vi "UHR-Fleezers Control (host) - Avogadro v1.vi"() -> ()   [LabVIEW 2014] (continued)
              }
            }
          }
          frame "Do nothing" {
          }
          frame "Initialize", Default {
            n3430 = Increment(x=w4831) -> (x+1=w4835:i32)
            n3431 = Select(t=1, s=w4824, f=w4835) -> (s? t:f=w4825:i32)
            n3432 = feedback #20(w4833) -> (w4839:dbl[])
            n3433 = Build Array (concatenate)(w4833, w4839) -> (w4832:dbl[])
            n3434 = Greater Or Equal?(x=w4825, y="Wait to get offset (n)") -> (x >= y?=w4828:bool)
            n3435 = Select(t=w4833, s=w4824, f=w4832) -> (s? t:f=w4834:dbl[])
            n3436 = feedback-in #20(w4834) -> ()
            n3437 = call-poly <vilib>:"Mean.vi"("X"=w4834) -> ("mean"=w4829:dbl)  [unwired: 1 out]
            n3438 = local write "Mean T1 Position\nto compare (nm)"(w4829) -> ()
            n3439 = case shown="True" w4824 {
              tunnel: w4827 -> [_ w4845]
              tunnel: w4826 -> [_ w4844]
              frame False {
              }
              frame True {
                w4841 = FALSE ("FPGA Trap Trig")
                n3440 = xnode "Read/Write Control"("FPGA VI Reference In"=w4845, "error in"=w4844, "FPGA Trap Trig"=w4841) -> ("FPGA VI Reference Out"=w4843:T41, "error out"=w4842:errorcluster)
                n3441 = xnode "Read/Write Control"("FPGA VI Reference In"=w4843, "error in"=w4842, "TTrig?"=w4841) -> ()  [unwired: 2 out]
              }
            }
            n3442 = Select(t="Wait for trigger", s=w4828, f="Initialize") -> (s? t:f=w4836:string)
            n3443 = case shown="True" w4828 {
              tunnel: w4829 -> [_ w4848]
              tunnel: w4827 -> [_ w4857]
              tunnel: w4826 -> [_ w4856]
              frame False {
                n3444 = local write "Waiting"(FALSE ("Waiting")) -> ()
                "Initializing" <- TRUE ("Initializing")
              }
              frame True {
                n3445 = local read "Threshold (nm)"() -> (w4860:dbl)
                n3446 = local read "AOM X Cal (nm/MHz)"() -> (w4859:dbl)
                n3447 = Add(x=w4848, y=w4860) -> (x+y=w4861:dbl)
                n3448 = Divide(x=w4861, y=w4859) -> (x/y=w4858:dbl)
                n3449 = call "IR AOM freq to word.vi"("Frequency In (MHz)"=w4858) -> ("Frequency Word Out (double)"=w4855:dbl)
                n3450 = local write "Initializing"(FALSE ("Initializing")) -> ()
                n3451 = local write "Waiting"(TRUE ("Waiting")) -> ()
                n3452 = To Quad Integer(1:w4855) -> (0:w4854:i64)
                n3453 = xnode "Read/Write Control"("FPGA VI Reference In"=w4857, "error in"=w4856, "FPGA TTrig Thresh"=w4854) -> ("FPGA VI Reference Out"=w4851:T41, "error out"=w4850:errorcluster)
                n3454 = xnode "Read/Write Control"("FPGA VI Reference In"=w4851, "error in"=w4850, "FPGA Trap Trig"=TRUE) -> ()  [unwired: 2 out]
              }
            }
          }
        }
      }
    }
    n3455 = feedback-in #18(w4440) -> ()
    n3456 = feedback-in #19(w4437) -> ()
    n3457 = xnode ("Read/Write Control")("FPGA VI Reference In"=w4251, "error in"=w4523) -> ("FPGA VI Reference Out"=w4325:T41, "error out"=w4425:errorcluster, "AI2 Y Sum Set 1"=w4572:i16, "AI2 Y Sum Set 2"=w4571:i16, "AI1 X Set 1"=w4463:fxp<+/-,16,1>, "AI1 X Set 2"=w4462:fxp<+/-,16,1>, "Trap Pos FB Int Signal"=→"Trap Pos FB Int Signal":fxp<+/-,24,9>, "Trap Pos FB Int-Norm Signal"=→"Trap Pos FB Int-Norm Signal":fxp<+/-,16,1>, "Trap Pos FB Action"=w4456:i64, "Scanning"=→"AOD Scanning":bool, "Scan I"=→"AOD Scan I":u64, "Scanning MCL"=w4574:bool, "Scan I (MCL)"=→"MCL Scan I":u64, "Green FB Sum"=w4536:i16, "Trap Pos FB Action"=w4423:i64, "TTrig Fin Thresh"=w4419:i64, "Red FB Intensity"=w4406:i16, "Blue Intensity"=w4401:i16, "BD1 Frequency Out 1"=w4342:u64)
    "MCL Scanning" <- w4574
    "Trap Pos FB Action" <- w4456
    n3458 = Divide(x=w4406, y=3276.7) -> (x/y=w4405:dbl)
    "Red laser intensity (V)" <- w4405
    n3459 = Divide(x=w4401, y=3276.7) -> (x/y=w4400:dbl)
    "Blue laser intensity (V)" <- w4400
    n3460 = Divide(x=w4536, y=3276.7) -> (x/y=w4404:dbl)
    "Green laser intensity (V)" <- w4404
    n3461 = local read "FB Trig Integrate"() -> (w4417:u32)
    n3462 = Divide(x=w4423, y=w4417) -> (x/y=w4416:dbl)
    "TTrig Sig (Int)" <- w4416
    n3463 = Bundle(w4404, w4405, w4400) -> (→"Fluorescence laser intensities plot":cluster{dbl, dbl, dbl})  [unwired: 1 in]
    n3464 = Divide(x=w4419, y=w4417) -> (x/y=w4414:dbl)
    "TTrig Fin Thresh (Int)" <- w4414
    n3465 = local read "AOM X Cal (nm/MHz)"() -> (w4422:dbl)
    n3466 = local read "AI2 (V)"() -> (w4573:cluster{"Set 1":dbl, "Set 2":dbl})
    n3467 = Bundle By Name(cluster=w4573, "Set 1"=w4572, "Set 2"=w4571) -> (w4344:cluster{"Set 1":dbl, "Set 2":dbl})
    n3468 = Divide(x=w4456, y=327.67) -> (x/y=→"Action (%)":dbl)
    n3469 = case shown="True" "Semi Passive Mode" {
      tunnel: w4323 -> [_ w4638]
      frame False {
      }
      frame True {
        n3470 = local read "Target Force (pN)"() -> (w4636:dbl)
        n3471 = Less?(x="Jump Force (pN)", y=w4636) -> (x < y?=w4634:bool)
        n3472 = case shown="False" w4634 {
          tunnel: "Jump Force (pN)" -> [w4644 w4647]
          tunnel: w4638 -> [w4643 w4646]
          tunnel: [w4642 w4645] -> w4637
          frame False {
            n3473 = Less?(x=w4644, y=w4643) -> (x < y?=w4642:bool)
          }
          frame True {
            n3474 = Greater?(x=w4647, y=w4646) -> (0:w4645:bool)
          }
        }
        n3475 = case shown="False" w4637 {
          frame False {
            n3476 = local read "Trap Pos. FB ON"() -> (w4639:bool)
            n3477 = case shown="False" w4639 {
              frame False {
              }
              frame True {
                n3478 = property on="Trap Pos. FB ON" class="Bool (strict)"("Val(Sgnl)"=FALSE) -> ()  [unwired: 2 in, 2 out]
              }
            }
          }
          frame True {
            n3479 = property on="Trap Pos. FB ON" class="Bool (strict)"("Val(Sgnl)"=TRUE) -> ()  [unwired: 2 in, 2 out]
          }
        }
      }
    }
    n3480 = local read "Trap X (AI1)"() -> (w4476:T15)
    n3481 = call "IR AOM word double to freq.vi"("Frequency Word In (double)"=w4414) -> ("Frequency Out (MHz)"=w4413:dbl)
    n3482 = call "IR AOM word double to freq.vi"("Frequency Word In (double)"=w4416) -> ("Frequency Out (MHz)"=w4415:dbl)
    n3483 = Divide(x=w4344, y=3276.7) -> (x/y=w4569:cluster{"Set 1":dbl, "Set 2":dbl})
    n3484 = Multiply(x=w4415, y=w4422) -> (x*y=w4421:dbl)
    "TTrig Sig (nm)" <- w4421
    n3485 = Multiply(x=w4413, y=w4422) -> (x*y=w4420:dbl)
    "TTrig Fin Thresh (nm)" <- w4420
    n3486 = local write "AI2 (V)"(w4569) -> ()
    n3487 = Bundle(cluster=w4476, "Trap 1"=w4463, "Trap 2"=w4462) -> (→"Trap X (AI1)":T15)
    n3488 = local read "Trap Pos. FB ON"() -> (w4330:bool)
    n3489 = local read "Dynamic Force FB (ronen)"() -> (w4331:bool)
    n3490 = Bundle(w4421, w4420) -> (→"TTrig":cluster{dbl, dbl})  [unwired: 1 in]
    n3491 = Compound Arithmetic op=AND(w4331, "Real time Offset file correction for setpoint", w4330) -> (w4332:bool)
    n3492 = case shown="True" w4332 {
      tunnel: w4342 -> [_ _]
      tunnel: w4328 -> [_ w4666]
      tunnel: w4325 -> [_ w4649]
      frame False {
      }
      frame True {
        # "Changed by Ronen - real time update of set point\naccording to offset file"
        n3493 = local read "T1 calibration"() -> (w4661:T9)
        n3494 = local read "Offset file step size"() -> (w4668:dbl)
        n3495 = local read "Setpoint offset\ncorrection values"() -> (w4665:dbl[])
        n3496 = Multiply(x="Target Force (pN)", y=2.0) -> (x*y=w4662:dbl)
        n3497 = local read "Negate Diff?"() -> (w4650:bool)
        n3498 = Unbundle By Name(w4661) -> ("alpha_x (nm/V)"=w4660:dbl, "kappa_x (pN/nm)"=w4659:dbl)
        n3499 = Divide(x=w4666, y=w4668) -> (x/y=w4669:dbl)
        n3500 = To Long Integer(number=w4669) -> (32bit integer=w4667:i32)
        n3501 = Index Array(array=w4665, index=w4667) -> (element=w4652:dbl)
        n3502 = Multiply(x=w4660, y=w4659) -> (x*y=w4658:dbl)
        n3503 = Select(t=1, s=w4650, f=-1) -> (s? t:f=w4653:i32)
        n3504 = Divide(x=w4662, y=w4658) -> (x/y=w4657:dbl)
        n3505 = Multiply(x=w4653, y=w4652) -> (x*y=w4651:dbl)
        n3506 = Add(x=w4657, y=w4651) -> (x+y=w4656:dbl)
        n3507 = To Fixed-Point(number=w4656) -> (fixed-point=w4648:fxp<+/-,16,1>)  [unwired: 1 in]
        "Actual Setpoint" <- w4648
        n3508 = xnode "Read/Write Control"("FPGA VI Reference In"=w4649, "Trap Pos. FB SP"=w4648) -> ()  [unwired: 1 in, 2 out]
      }
    }
    n3509 = local read "All FB On/Off"() -> (w4343:bool)
    n3510 = case shown="True" w4343 {
      tunnel: w4344 -> [_ w4672]
      frame False {
      }
      frame True {
        n3511 = Divide(x=w4672, y=3276.7) -> (x/y=w4670:cluster{"Set 1":dbl, "Set 2":dbl})
        n3512 = Unbundle By Name(w4670) -> ("Set 1"=w4677:dbl, "Set 2"=w4676:dbl)
        n3513 = Greater?(x=w4677, y="Feedback Auto-Off threshold") -> (0:w4675:bool)
        n3514 = Greater?(x=w4676, y="Feedback Auto-Off threshold") -> (0:w4674:bool)
        n3515 = Or(x=w4675, y=w4674) -> (x .or. y?=w4673:bool)
        n3516 = case shown="True" w4673 {
          frame False {
          }
          frame True {
            n3517 = property on="All FB On/Off" class="Bool (strict)"("Val(Sgnl)"=FALSE) -> ()  [unwired: 2 in, 2 out]
          }
        }
      }
    }
    n3518 = flat-sequence "To save data" {
      tunnel: [w5430] -> w4592
      tunnel: [w5431] -> w4591
      tunnel: w4554 -> [w5424]
      tunnel: w4284 -> [w5428]
      tunnel: ["Save Calibration"] -> w4566
      tunnel: w4314 -> [w5427]
      tunnel: [w5420] -> w4563
      tunnel: [w5417] -> w4562
      tunnel: [w5414] -> w4561
      tunnel: w4553 -> [w5416]
      tunnel: w4250 -> [w5410]
      tunnel: [w5410] -> w4517
      tunnel: ["Start Saving"] -> w4497
      tunnel: [w5405] -> w4446
      tunnel: [w5404] -> w4445
      tunnel: [w5401] -> w4348
      tunnel: [w5397] -> w4336
      tunnel: w4592 -> [w5742]
      tunnel: w4591 -> [w5741]
      tunnel: w4315 -> [w5740]
      tunnel: w4566 -> [w5739]
      tunnel: w4563 -> [w5737]
      tunnel: w4562 -> [w5736]
      tunnel: w4561 -> [w5735]
      tunnel: w4307 -> [w5734]
      tunnel: w4313 -> [w5733]
      tunnel: w4517 -> [w5732]
      tunnel: w4497 -> [w5731]
      tunnel: w4355 -> [w5730]
      tunnel: w4396 -> [w5729]
      tunnel: w4446 -> [w5728]
      tunnel: w4445 -> [w5727]
      tunnel: w4444 -> [w5726]
      tunnel: w4256 -> [w5725]
      tunnel: w4312 -> [w5724]
      tunnel: w4348 -> [w5723]
      tunnel: w4336 -> [w5722]
      frame #0 {
        # "Changed by Ronen - we don't have a database so we disabled this"
        n3519 = Or(x="Save N Sets", y="Start Saving") -> (x .or. y?=w5411:bool)
        n3520 = To Double Precision Float(number=w5427) -> (double precision float=w5421:dbl)
        n3521 = Build Array(w5411, "Save Calibration", w5424, w5416, "Flow Cal") -> (w5426:bool[])
        n3522 = Compound Arithmetic op=OR("Save Calibration", w5424, w5411, w5416, "Flow Cal") -> (w5429:bool)
        n3523 = Boolean Array To Number(Boolean array=w5426) -> (number=w5423:u32)
        n3524 = feedback #21(FALSE ("Save APD Data\nwith Trap Data")) -> (w5406:bool)
        n3525 = feedback #22(refnum<k0> refnum) -> (w5432:refnum<file>)
        n3526 = feedback #23(FALSE ("Save APD Data\nwith Trap Data")) -> (w5415:bool)
        n3527 = feedback #24(0) -> (w5434:i32)
        n3528 = feedback #25() -> (w5422:u32)  [unwired: 1 out]
        n3529 = feedback #26(refnum<k0> refnum) -> (w5402:refnum<file>)
        n3530 = feedback #27(refnum<k0> refnum) -> (w5408:refnum<file>)
        n3531 = feedback #28(refnum<k0> refnum) -> (w5398:refnum<file>)
        n3532 = feedback #29(refnum<k0> refnum) -> (w5418:refnum<file>)
        n3533 = case shown="True" w5429 {
          tunnel: [w5443 1] -> w5430
          tunnel: w5434 -> [w5445 _]
          tunnel: [w5444 w5477] -> w5431
          tunnel: w5432 -> [w5444 _]
          tunnel: w5428 -> [_ w5495]
          tunnel: w5421 -> [_ w5493]
          tunnel: w5423 -> [_ w5496]
          tunnel: [w5442 w5476] -> w5420
          tunnel: w5422 -> [w5442 _]
          tunnel: [w5441 w5474] -> w5417
          tunnel: w5418 -> [w5441 _]
          tunnel: [w5440 w5473] -> w5414
          tunnel: w5415 -> [w5440 _]
          tunnel: "Start Saving" -> [_ w5471]
          tunnel: w5410 -> [_ w5470]
          tunnel: [w5439 w5463] -> w5404
          tunnel: w5408 -> [w5439 _]
          tunnel: [w5438 w5462] -> w5405
          tunnel: w5406 -> [w5438 _]
          tunnel: [w5437 w5448] -> w5401
          tunnel: w5402 -> [w5437 _]
          tunnel: [w5436 w5446] -> w5397
          tunnel: w5398 -> [w5436 _]
          frame False {
            n3534 = Increment(x=w5445) -> (x+1=w5443:i32)
          }
          frame True {
            w5447 = FALSE ("Start Saving")
            w5472 = 10.0  # File Version
            w5479 = FALSE ("prepend array or string size? (T)")
            w5478 = T45."big-endian, network order" ("byte order (0:big-endian, network order)")
            # "Ronen Changed the create file - changed data folder to c:\\Data"
            # "Save trap position\ndata"
            n3535 = Array Size(array=w5470) -> (size(s)=w5469:i32)
            n3536 = To Double Precision Float(number=w5469) -> (double precision float=w5468:dbl)
            n3537 = local read "BD 1 Frequency 1 (MHz)"() -> (w5492:dbl)
            n3538 = local read "BD 2 Frequency 1 (MHz)"() -> (w5491:dbl)
            n3539 = local read "BD 1 Frequency 2 (MHz)"() -> (w5490:dbl)
            n3540 = local read "BD 2 Frequency 2 (MHz)"() -> (w5489:dbl)
            n3541 = local read "BD 1 Frequency 3 (MHz)"() -> (w5488:dbl)
            n3542 = local read "BD 2 Frequency 3 (MHz)"() -> (w5487:dbl)
            n3543 = local write "Flow Cal"(w5447) -> ()
            n3544 = local write "Save Calibration"(w5447) -> ()
            n3545 = local write "Start Saving"(w5447) -> ()
            n3546 = Build Array("Save APD Data\nwith Trap Data", "Save Trap Pos. Data") -> (w5465:bool[])
            n3547 = Boolean Array To Number(Boolean array=w5465) -> (number=w5464:u32)
            n3548 = Build Array(w5492, w5491, w5490, w5489, w5488, w5487) -> (w5486:dbl[])
            n3549 = case shown="4" w5496 {
              tunnel: w5495 -> [w5596 w5623 w5639 w5677 w5714]
              tunnel: w5468 -> [w5601 w5630 w5659 w5696 w5719]
              tunnel: w5493 -> [w5600 w5629 w5658 w5695 w5718]
              tunnel: [w5597 w5625 w5650 w5687 w5715] -> w5484
              tunnel: [w5588 "Cal sets to save" w5640 w5678 w5701] -> w5476
              tunnel: w5486 -> [w5598 w5626 w5652 w5689 w5716]
              tunnel: "Save APD Data\nwith Trap Data" -> [w5595 w5612 w5636 w5675 w5713]
              tunnel: [w5595 w5610 w5636 w5675 w5713] -> w5473
              tunnel: w5472 -> [w5591 w5619 w5634 w5673 w5709]
              tunnel: w5471 -> [w5590 _ _ _ _]
              tunnel: [w5581 w5618 w5633 w5663 w5708] -> w5462
              tunnel: "Save Trap Pos. Data" -> [w5581 w5617 w5633 w5663 w5708]
              tunnel: w5464 -> [w5580 w5616 w5632 w5662 w5707]
              frame 1, Default {
                # "timeseries"
                n3550 = case shown="True" "Profile" {
                  tunnel: [w5604 w5608] -> w5585
                  tunnel: [w5604 w5607] -> w5584
                  tunnel: [w5604 w5606] -> w5583
                  tunnel: [w5604 w5605] -> w5582
                  frame False {
                    w5604 = 0.0 ("f")
                  }
                  frame True {
                    n3551 = local read "Current Position"() -> (w5609:cluster{dbl, dbl, dbl})
                    n3552 = local read "Y change (mm)"() -> (w5605:dbl)
                    n3553 = Unbundle(w5609) -> (w5608:dbl, w5607:dbl, w5606:dbl)
                  }
                }
                n3554 = local read "Save ave N"() -> (w5603:dbl)
                n3555 = Multiply(x=w5603, y=w5596) -> (x*y=w5602:dbl)
                n3556 = To Double Precision Float(number=w5580) -> (double precision float=w5594:dbl)
                n3557 = Build Array(w5591, w5596, w5602, w5601, w5600, 0.0 ("f")) -> (w5599:dbl[])
                n3558 = Build Array(w5594, w5585, w5584, w5583, w5582) -> (w5592:dbl[])
                n3559 = Select(t=u32 4000000000, s=w5590, f="N sets to save") -> (s? t:f=w5588:u32)
                n3560 = Build Array (concatenate)(w5599, w5598, w5592) -> (w5597:dbl[])
              }
              frame 2 {
                w5621 = 0.0 ("f")
                w5611 = FALSE ("Save APD Data\nwith Trap Data")
                # "For diagnostics save trap position\ndata during cal"
                # "calibration"
                n3561 = Boolean To (0,1)(Boolean=w5611) -> (0, 1=w5615:i16)
                n3562 = Select(t=w5612, s="Save trap pos with cal", f=w5611) -> (s? t:f=w5610:bool)
                n3563 = Select(t=w5617, s="Save trap pos with cal", f=w5611) -> (s? t:f=w5618:bool)
                n3564 = Select(t=w5616, s="Save trap pos with cal", f=w5615) -> (s? t:f=w5614:u32)
                n3565 = To Double Precision Float(number=w5614) -> (double precision float=w5622:dbl)
                n3566 = Build Array(w5619, w5623, w5623, w5630, w5629, 1.0 ("t")) -> (w5627:dbl[])
                n3567 = Build Array(w5622, w5621, w5621, w5621, w5621) -> (w5620:dbl[])
                n3568 = Build Array (concatenate)(w5627, w5626, w5620) -> (w5625:dbl[])
                "Calibrating Trap..." <- TRUE ("Calibrating...")
              }
              frame 4 {
                w5637 = 0.0 ("f")
                # "scan dir (x/y = 0/1)"
                # "cycles/step"
                # "n scans (f/b)"
                # "steps"
                # "freq. range"
                # "AOD raster scan"
                n3569 = local read "Number of F/B Scans (AOD)"() -> (w5644:u16)
                n3570 = local read "Cycles/step (AOD)"() -> (w5646:u64)
                n3571 = local read "Scan Range (MHz)"() -> (w5649:dbl)
                n3572 = local read "Scan steps (AOD)"() -> (w5648:u64)
                n3573 = local read "Scan BD"() -> (w5656:bool)
                n3574 = local read "Save ave N"() -> (w5661:dbl)
                n3575 = Boolean To (0,1)(Boolean=w5656) -> (0, 1=w5655:i16)
                n3576 = To Double Precision Float(number=w5644) -> (double precision float=w5643:dbl)
                n3577 = To Double Precision Float(number=w5648) -> (double precision float=w5647:dbl)
                n3578 = To Double Precision Float(number=w5646) -> (double precision float=w5645:dbl)
                n3579 = To Double Precision Float(number=w5655) -> (double precision float=w5654:dbl)
                n3580 = Multiply(x=w5661, y=w5639) -> (x*y=w5660:dbl)
                n3581 = To Double Precision Float(number=w5632) -> (double precision float=w5638:dbl)
                n3582 = Build Array(w5638, w5637, w5637, w5637, w5637) -> (w5635:dbl[])
                n3583 = local read "N sets should be saved"() -> (w5641:dbl)
                n3584 = Build Array(w5654, w5649, w5647, w5645, w5643) -> (w5651:dbl[])
                n3585 = Build Array(w5634, w5639, w5660, w5659, w5658, 2.0 ("t")) -> (w5653:dbl[])
                n3586 = Round Toward +Infinity(x=w5641) -> (ceil(x): smallest int >= x=w5642:dbl)
                n3587 = Build Array (concatenate)(w5653, w5652, w5635, w5651) -> (w5650:dbl[])
                n3588 = To Unsigned Long Integer(number=w5642) -> (unsigned 32bit integer=w5640:u32)
              }
              frame 8 {
                w5670 = 0.0 ("f")
                # "MCL raster scan"
                n3589 = local read "Number of scans (MCL)"() -> (w5665:u64)
                n3590 = local read "2D or 1D Scan"() -> (w5667:bool)
                n3591 = local read "Scan lines (y)"() -> (w5664:u64)
                n3592 = local read "Scan Range (V)\n(of steps)"() -> (w5686:dbl)
                n3593 = local read "Fast Scan Dir"() -> (w5693:bool)
                n3594 = local read "Cycles/step (MCL)"() -> (w5683:u64)
                n3595 = local read "Scan steps (MCL)"() -> (w5685:u64)
                n3596 = Select(t=w5664, s=w5667, f=w5665) -> (s? t:f=w5666:u64)
                n3597 = Boolean To (0,1)(Boolean=w5667) -> (0, 1=w5669:i16)
                n3598 = local read "Save ave N"() -> (w5698:dbl)
                n3599 = local read "Initial X"() -> (w5672:dbl)
                n3600 = local read "Initial Y"() -> (w5671:dbl)
                n3601 = To Double Precision Float(number=w5669) -> (double precision float=w5668:dbl)
                n3602 = Boolean To (0,1)(Boolean=w5693) -> (0, 1=w5692:i16)
                n3603 = To Double Precision Float(number=w5666) -> (double precision float=w5681:dbl)
                n3604 = To Double Precision Float(number=w5685) -> (double precision float=w5684:dbl)
                n3605 = To Double Precision Float(number=w5683) -> (double precision float=w5682:dbl)
                n3606 = To Double Precision Float(number=w5692) -> (double precision float=w5691:dbl)
                n3607 = Multiply(x=w5698, y=w5677) -> (x*y=w5697:dbl)
                n3608 = To Double Precision Float(number=w5662) -> (double precision float=w5676:dbl)
                n3609 = local read "N sets should be saved (MCL)"() -> (w5679:dbl)
                n3610 = Build Array(w5676, w5668, w5670, w5670, w5670) -> (w5674:dbl[])
                n3611 = Build Array(w5691, w5686, w5684, w5682, w5681, w5672, w5671) -> (w5688:dbl[])
                n3612 = Build Array(w5673, w5677, w5697, w5696, w5695, 3.0 ("t")) -> (w5690:dbl[])
                n3613 = Round Toward +Infinity(x=w5679) -> (ceil(x): smallest int >= x=w5680:dbl)
                n3614 = Build Array (concatenate)(w5690, w5689, w5674, w5688) -> (w5687:dbl[])
                n3615 = To Unsigned Long Integer(number=w5680) -> (unsigned 32bit integer=w5678:u32)
              }
              frame 16 {
                w5700 = 0.0
                # "Flow calibration - added by Ronen: Number\nof saved sets is distance (1 mm) divided by \nspeed +1.5 spare second divided by the time of\nset measurement, 0.2 sec for 2 set interlace"
                # "timeseries"
                n3616 = local read "Save ave N"() -> (w5721:dbl)
                n3617 = Reciprocal(x=0.0) -> (1/x=w5706:dbl)
                n3618 = Add(x=w5706, y=1.5) -> (x+y=w5704:dbl)
                n3619 = Multiply(x=w5721, y=w5714) -> (x*y=w5720:dbl)
                n3620 = Divide(x=w5704, y=0.2) -> (x/y=w5702:dbl)
                n3621 = To Double Precision Float(number=w5707) -> (double precision float=w5712:dbl)
                n3622 = To Unsigned Long Integer(number=w5702) -> (unsigned 32bit integer=w5701:u32)
                n3623 = Build Array(w5709, w5714, w5720, w5719, w5718, 4.0 ("f")) -> (w5717:dbl[])
                n3624 = Build Array(w5712, w5700, w5700, w5700, w5700) -> (w5710:dbl[])
                n3625 = Build Array (concatenate)(w5717, w5716, w5710) -> (w5715:dbl[])
              }
            }
            n3626 = local read "Index"() -> (w5501:dbl)
            n3627 = call "Create new save file.vi"("Insert"="", "Ext"=".dat", "Index In"=w5501) -> ("Path Out"=w5450:path, "Index Out"=w5475:dbl)
            n3628 = local write "Save file name"(w5450) -> ()
            n3629 = local write "Index"(w5475) -> ()
            n3630 = local write "Save index"(w5475) -> ()
            n3631 = case shown="True" "Save Event Log?" {
              tunnel: w5450 -> [_ w5515]
              tunnel: [refnum<k0> refnum w5514] -> w5448
              frame False {
              }
              frame True {
                (unwired) FALSE ("prepend array or string size? (T)")
                n3632 = Path To String(path=w5515) -> (string=w5526:string)
                n3633 = String Length(string=w5526) -> (length=w5525:i32)
                n3634 = Subtract(x=w5525, y=4) -> (x-y=w5523:i32)
                n3635 = String Subset(string=w5526, length (rest)=w5523) -> (substring=w5522:string)  [unwired: 1 out]
                n3636 = Concatenate Strings(w5522, "_log.txt" ("string")) -> (w5520:string)
                n3637 = String To Path(string=w5520) -> (path=w5516:path)
                n3638 = Open/Create/Replace File(file path (use dialog)=w5516, operation (0:open)=T44."create", access (0:read/write)=enum16{"read/write", "read-only", "write-only"}."write-only") -> (refnum out=w5517:refnum<file>)  [unwired: 1 in, 4 out]
                n3639 = Deny Access(7:w5517) -> (3:w5514:refnum<file>)  [unwired: 1 in, 2 out]
                n3640 = call "write to event log.vi"("log file ref"=w5514, "time"=0.0, "input string"="start log") -> ()  [unwired: 8 in]
              }
            }
            "log file ref" <- w5448
            n3641 = Array Size(array=w5484) -> (size(s)=w5485:i32)
            n3642 = Open/Create/Replace File(file path (use dialog)=w5450, operation (0:open)=T44."create", access (0:read/write)=enum16{"read/write", "read-only", "write-only"}."write-only") -> (refnum out=w5498:refnum<file>)  [unwired: 1 in, 4 out]
            n3643 = local write "Saving..."(TRUE ("Saving...")) -> ()
            n3644 = To Double Precision Float(number=w5485) -> (double precision float=w5483:dbl)
            n3645 = String Length(string="Comment (data description)") -> (length=w5482:i32)
            n3646 = To Double Precision Float(number=w5482) -> (double precision float=w5481:dbl)
            n3647 = Deny Access(7:w5498) -> (3:w5497:refnum<file>)  [unwired: 1 in, 2 out]
            n3648 = Build Array (concatenate)(w5483, w5484, w5481) -> (w5460:dbl[])
            n3649 = case "If fluorescence data to be saved" shown="True" w5473 {
              tunnel: w5450 -> [_ w5579]
              tunnel: [w5549 w5562] -> w5474
              tunnel: [w5549 w5550] -> w5446
              frame False {
                w5549 = refnum<k0> refnum
              }
              frame True {
                w5561 = 0.0
                w5554 = T44."create" ("operation (0:open)")
                w5555 = enum16{"read/write", "read-only", "write-only"}."write-only" ("access (0:read/write)")
                n3650 = local read "APD Integration Time (s)"() -> (w5567:dbl)
                n3651 = local read "N APD Samp/step"() -> (w5560:dbl)
                n3652 = local read "Number of APDs"() -> (w5559:u8)
                n3653 = Path To String(path=w5579) -> (string=w5578:string)
                n3654 = String Length(string=w5578) -> (length=w5577:i32)
                n3655 = Subtract(x=w5577, y=4) -> (x-y=w5575:i32)
                n3656 = String Subset(string=w5578, length (rest)=w5575) -> (substring=w5558:string)  [unwired: 1 out]
                n3657 = Build Array(w5567, w5560, w5559, w5561, w5561, w5561, w5561, w5561) -> (w5564:dbl[])
                n3658 = Concatenate Strings(w5558, "_green.dat") -> (w5556:string)
                n3659 = Concatenate Strings(w5558, "_fl.dat" ("string")) -> (w5573:string)
                n3660 = Array Size(array=w5564) -> (size(s)=w5566:i32)
                n3661 = String To Path(string=w5573) -> (path=w5571:path)
                n3662 = Open/Create/Replace File(file path (use dialog)=w5571, operation (0:open)=w5554, access (0:read/write)=w5555) -> (refnum out=w5572:refnum<file>)  [unwired: 1 in, 4 out]
                n3663 = Deny Access(7:w5572) -> (3:w5568:refnum<file>)  [unwired: 1 in, 2 out]
                n3664 = String To Path(string=w5556) -> (path=w5553:path)
                n3665 = To Double Precision Float(number=w5566) -> (double precision float=w5565:dbl)
                n3666 = Build Array (concatenate)(w5565, w5564) -> (w5563:dbl[])
                n3667 = Write to Binary File(file (use dialog)=w5568, data=w5563, 5:FALSE ("prepend array or string size? (T)"), 9:T45."big-endian, network order" ("byte order (0:big-endian, network order)")) -> (refnum out=w5562:refnum<file>)  [unwired: 1 in, 3 out]
                n3668 = Open/Create/Replace File(file path (use dialog)=w5553, operation (0:open)=w5554, access (0:read/write)=w5555) -> (refnum out=w5551:refnum<file>, error out=w5552:errorcluster)  [unwired: 3 in, 1 out]
                n3669 = Deny Access(4:w5552, 7:w5551) -> (3:w5550:refnum<file>)  [unwired: 1 in, 1 out]
              }
            }
            n3670 = case shown="True" w5462 {
              tunnel: w5450 -> [_ w5534]
              tunnel: [refnum<k0> refnum w5533] -> w5463
              frame False {
              }
              frame True {
                w5529 = 0.0 ("element")
                n3671 = Path To String(path=w5534) -> (string=w5548:string)
                n3672 = Build Array(w5529, w5529, w5529, w5529, w5529, w5529, w5529, w5529) -> (w5530:dbl[])
                n3673 = String Length(string=w5548) -> (length=w5547:i32)
                n3674 = Subtract(x=w5547, y=4) -> (x-y=w5545:i32)
                n3675 = Array Size(array=w5530) -> (size(s)=w5532:i32)
                n3676 = String Subset(string=w5548, length (rest)=w5545) -> (substring=w5544:string)  [unwired: 1 out]
                n3677 = To Double Precision Float(number=w5532) -> (double precision float=w5531:dbl)
                n3678 = Concatenate Strings(w5544, "_pos.dat" ("string")) -> (w5542:string)
                n3679 = Build Array (concatenate)(w5531, w5530) -> (w5528:dbl[])
                n3680 = String To Path(string=w5542) -> (path=w5538:path)
                n3681 = Open/Create/Replace File(file path (use dialog)=w5538, operation (0:open)=T44."create", access (0:read/write)=enum16{"read/write", "read-only", "write-only"}."write-only") -> (refnum out=w5539:refnum<file>)  [unwired: 1 in, 4 out]
                n3682 = Deny Access(7:w5539) -> (3:w5535:refnum<file>)  [unwired: 1 in, 2 out]
                n3683 = Write to Binary File(file (use dialog)=w5535, data=w5528, 5:FALSE ("prepend array or string size? (T)"), 9:T45."big-endian, network order" ("byte order (0:big-endian, network order)")) -> (refnum out=w5533:refnum<file>)  [unwired: 1 in, 3 out]
              }
            }
            n3684 = Write to Binary File(file (use dialog)=w5497, data=w5460, 5:w5479, 9:w5478) -> (refnum out=w5480:refnum<file>)  [unwired: 1 in, 3 out]
            n3685 = Write to Binary File(file (use dialog)=w5480, data="Comment (data description)", 5:w5479, 9:w5478) -> (refnum out=w5477:refnum<file>)  [unwired: 1 in, 3 out]
            n3686 = local read "connection reference"() -> (w5461:T24)
            n3687 = Bundle("Comment (data description)"="Comment (data description)", "Channel 1 Buffer"="Channel 1 Buffer", "Channel 2 Buffer"="Channel 2 Buffer", "Channel 3 Buffer"="Channel 3 Buffer", "Title"="Title", "DNA Construct"="DNA Construct", "Bead diameter"="Bead diameter", "Name"="Name") -> (w5451:T67)  [unwired: 1 in]
            n3688 = disable-structure shown="Disabled" {
              disable-tunnel: w5461 -> [w5509 _]
              disable-tunnel: w5460 -> [w5507 _]
              disable-tunnel: w5451 -> [w5506 _]
              disable-tunnel: w5450 -> [w5505 _]
              frame Disabled {
                n3689 = call "MattFileCreator-v9.vi"("Comments"=w5506, "Input Array"=w5507, "File path"=w5505, "table"="labview", "connection reference"=w5509) -> ("connection reference out"=w5508:T24)  [unwired: 5 in, 1 out]
                n3690 = local write "connection reference"(w5508) -> ()
              }
              frame Enabled {
              }
            }
          }
        }
        n3691 = feedback-in #21(w5405) -> ()
        n3692 = feedback-in #22(w5431) -> ()
        n3693 = feedback-in #23(w5414) -> ()
        n3694 = feedback-in #24(w5430) -> ()
        n3695 = feedback-in #25(w5420) -> ()
        n3696 = feedback-in #26(w5401) -> ()
        n3697 = feedback-in #27(w5404) -> ()
        n3698 = feedback-in #28(w5397) -> ()
        n3699 = feedback-in #29(w5417) -> ()
      }
      frame #1 {
        n3700 = local read "Saving..."() -> (w5738:bool)
        n3701 = case shown="True" w5738 {
          tunnel: w5742 -> [_ w5756]
          tunnel: w5741 -> [_ w5770]
          tunnel: w5740 -> [_ w5766]
          tunnel: w5739 -> [_ w5765]
          tunnel: w5737 -> [_ w5764]
          tunnel: w5736 -> [_ w5759]
          tunnel: w5735 -> [_ w5758]
          tunnel: w5734 -> [_ w5757]
          tunnel: w5733 -> [_ w5755]
          tunnel: w5732 -> [_ w5753]
          tunnel: w5731 -> [_ w5752]
          tunnel: w5730 -> [_ w5751]
          tunnel: w5729 -> [_ w5750]
          tunnel: w5728 -> [_ w5749]
          tunnel: w5727 -> [_ w5748]
          tunnel: w5726 -> [_ w5747]
          tunnel: w5725 -> [_ w5746]
          tunnel: w5724 -> [_ w5745]
          tunnel: w5723 -> [_ w5744]
          tunnel: w5722 -> [_ w5743]
          frame False {
          }
          frame True {
            n3702 = Multiply(x=w5756, y=w5755) -> (x*y=→"Time (s)":dbl)
            n3703 = Less Or Equal?(x=w5756, y=w5764) -> (x <= y?=w5768:bool)
            n3704 = Compound Arithmetic op=OR("Stop Saving", "Abort save 2") -> (w5760:bool)
            n3705 = Not(x=w5760) -> (.not. x?=w5769:bool)
            n3706 = And(x=w5768, y=w5769) -> (x .and. y?=w5767:bool)
            n3707 = case shown="True" w5767 {
              tunnel: w5770 -> [w5780 w5881]
              tunnel: [0.0 w5884] -> w5763
              tunnel: w5756 -> [_ w5882]
              tunnel: w5764 -> [_ w5883]
              tunnel: w5766 -> [_ w5878]
              tunnel: w5765 -> [_ _]
              tunnel: w5759 -> [w5778 w5871]
              tunnel: w5758 -> [w5777 w5872]
              tunnel: w5757 -> [_ w5870]
              tunnel: w5753 -> [_ w5869]
              tunnel: w5752 -> [_ w5787]
              tunnel: w5751 -> [_ w5862]
              tunnel: w5750 -> [_ w5809]
              tunnel: w5749 -> [w5774 w5826]
              tunnel: w5748 -> [w5775 w5825]
              tunnel: w5747 -> [_ w5822]
              tunnel: w5746 -> [_ w5820]
              tunnel: w5745 -> [_ w5786]
              tunnel: w5744 -> [w5773 _]
              tunnel: w5743 -> [w5771 w5785]
              frame False {
                w5776 = FALSE
                n3708 = Close File(refnum=w5780) -> ()  [unwired: 1 in, 2 out]
                n3709 = case shown="True" w5777 {
                  tunnel: w5778 -> [_ w5784]
                  tunnel: w5771 -> [_ w5783]
                  frame False {
                  }
                  frame True {
                    n3710 = Close File(refnum=w5784) -> ()  [unwired: 1 in, 2 out]
                    n3711 = Close File(refnum=w5783) -> ()  [unwired: 1 in, 2 out]
                  }
                }
                n3712 = case shown="True" w5774 {
                  tunnel: w5775 -> [_ w5782]
                  frame False {
                  }
                  frame True {
                    n3713 = Close File(refnum=w5782) -> ()  [unwired: 1 in, 2 out]
                  }
                }
                n3714 = local read "Save Event Log?"() -> (w5772:bool)
                n3715 = case shown="True" w5772 {
                  tunnel: w5773 -> [_ w5781]
                  frame False {
                  }
                  frame True {
                    n3716 = Close File(refnum=w5781) -> ()  [unwired: 1 in, 2 out]
                  }
                }
                n3717 = local write "Raster Scanning..."(w5776) -> ()
                n3718 = local write "Calibrating Trap..."(w5776) -> ()
                n3719 = call <vilib>:"Beep.vi"() -> ()  [unwired: 3 in, 9 out]
                n3720 = local write "Stop Saving"(w5776) -> ()
                "Saving..." <- w5776
              }
              frame True {
                n3721 = local read "Calibrating Trap..."() -> (w5873:bool)
                n3722 = case "Write fl. data" shown="True" w5872 {
                  tunnel: w5871 -> [_ w5914]
                  tunnel: w5870 -> [_ w5913]
                  tunnel: w5785 -> [_ w5907]
                  frame False {
                  }
                  frame True {
                    w5906 = FALSE ("prepend array or string size? (T)")
                    w5908 = T45."big-endian, network order" ("byte order (0:big-endian, network order)")
                    n3723 = property on="Green Laser ON" class="Bool (strict)"() -> ("Value"=w5912:bool)  [unwired: 2 in, 2 out]
                    n3724 = property on="Green Intensity % (FB OFF)" class="DigNum (strict)"() -> ("Value"=w5911:dbl)  [unwired: 2 in, 2 out]
                    n3725 = Boolean To (0,1)(Boolean=w5912) -> (0, 1=w5910:i16)
                    n3726 = Multiply(x=w5910, y=w5911) -> (x*y=w5909:dbl)
                    n3727 = Write to Binary File(file (use dialog)=w5914, data=w5913, 5:w5906, 9:w5908) -> ()  [unwired: 1 in, 4 out]
                    n3728 = Write to Binary File(file (use dialog)=w5907, data=w5909, 5:w5906, 9:w5908) -> ()  [unwired: 2 in, 3 out]
                  }
                }
                n3729 = Greater?(x="Save ave N", y=1.0) -> (0:w5876:bool)
                n3730 = Not(x=w5873) -> (.not. x?=w5875:bool)
                n3731 = And(x=w5875, y=w5876) -> (x .and. y?=w5823:bool)
                n3732 = case shown="True" w5823 {
                  tunnel: w5822 -> [w5887 w5898]
                  tunnel: [w5887 w5890] -> w5821
                  tunnel: "Save ave N" -> [_ w5891]
                  frame False {
                  }
                  frame True {
                    w5888 = 2 ("dimension size")
                    n3733 = Array Size(array=w5898) -> (size(s)=w5892:i32)
                    n3734 = Divide(x=w5892, y=w5888) -> (x/y=w5896:dbl)
                    n3735 = Reshape Array(w5898, w5896, w5888) -> (w5897:u64[][])
                    n3736 = Transpose 2D Array(2D array=w5897) -> (transposed array=w5895:u64[][])
                    n3737 = for {
                      tunnel: w5895 -> [w5900] mode=indexing
                      tunnel: [w5899] -> w5889 mode=indexing
                      tunnel: w5891 -> [w5901]
                      workers-P: _ -> [_]
                      n3738 = call "downsample 1D array - U64.vi"("Ave N"=w5901, "Array In"=w5900) -> ("Array Out"=w5899:u64[])  [unwired: 1 in]
                    }
                    n3739 = Transpose 2D Array(2D array=w5889) -> (transposed array=w5894:u64[][])
                    n3740 = Divide(x=w5892, y=w5891) -> (x/y=w5893:dbl)
                    n3741 = Reshape Array(w5894, w5893) -> (w5890:u64[])
                  }
                }
                n3742 = case shown="True" w5823 {
                  tunnel: w5878 -> [w5915 w5927]
                  tunnel: [w5915 w5919] -> w5874
                  tunnel: "Save ave N" -> [_ w5920]
                  tunnel: w5869 -> [_ w5918]
                  frame False {
                  }
                  frame True {
                    n3743 = Array Size(array=w5927) -> (size(s)=w5921:i32)
                    n3744 = Array Size(array=w5918) -> (size(s)=w5917:i32)
                    n3745 = Divide(x=w5921, y=w5917) -> (x/y=w5925:dbl)
                    n3746 = Reshape Array(w5927, w5925, w5917) -> (w5926:i16[][])
                    n3747 = Transpose 2D Array(2D array=w5926) -> (transposed array=w5924:i16[][])
                    n3748 = for {
                      tunnel: w5924 -> [w5930] mode=indexing
                      tunnel: [w5929] -> w5916 mode=indexing
                      tunnel: w5920 -> [w5928]
                      workers-P: _ -> [_]
                      n3749 = call "downsample 1D array - I16 to F32.vi"("Ave N"=w5928, "Array In"=w5930) -> ("Array Out"=w5929:sgl[])  [unwired: 1 in]
                    }
                    n3750 = Transpose 2D Array(2D array=w5916) -> (transposed array=w5923:sgl[][])
                    n3751 = Divide(x=w5921, y=w5920) -> (x/y=w5922:dbl)
                    n3752 = Reshape Array(w5923, w5922) -> (w5919:sgl[])
                  }
                }
                n3753 = Index Array(array=w5809, index=2) -> (element=w5810:waveform(dbl))
                n3754 = Index Array(array=w5809, index=1) -> (element=w5843:waveform(dbl))
                n3755 = Index Array(array=w5809, index=0) -> (element=w5845:waveform(dbl))
                n3756 = Unbundle By Name(w5810) -> ("Y"=w5812:dbl[])
                n3757 = Unbundle By Name(w5843) -> ("Y"=w5847:dbl[])
                n3758 = Unbundle By Name(w5845) -> ("Y"=w5855:dbl[])
                n3759 = case "Write trap pos. data" shown="True" w5826 {
                  tunnel: w5825 -> [_ w5903]
                  tunnel: w5821 -> [_ w5902]
                  frame False {
                  }
                  frame True {
                    n3760 = Write to Binary File(file (use dialog)=w5903, data=w5902, 5:FALSE ("prepend array or string size? (T)"), 9:T45."big-endian, network order" ("byte order (0:big-endian, network order)")) -> ()  [unwired: 1 in, 4 out]
                  }
                }
                n3761 = Write to Binary File(file (use dialog)=w5881, data=w5874, 5:FALSE ("prepend array or string size? (T)"), 9:T45."big-endian, network order" ("byte order (0:big-endian, network order)")) -> ()  [unwired: 1 in, 4 out]
                n3762 = feedback #30(w5812) -> (w5813:dbl[])
                n3763 = Build Array (concatenate)(w5813, w5812) -> (w5808:dbl[])
                n3764 = Select(t=w5812, s=w5787, f=w5808) -> (s? t:f=w5798:dbl[])
                n3765 = feedback-in #30(w5798) -> ()
                n3766 = feedback #31(w5847) -> (w5849:dbl[])
                n3767 = Build Array (concatenate)(w5849, w5847) -> (w5848:dbl[])
                n3768 = Select(t=w5847, s=w5787, f=w5848) -> (s? t:f=w5837:dbl[])
                n3769 = feedback-in #31(w5837) -> ()
                n3770 = feedback #32(w5855) -> (w5868:dbl[])
                n3771 = Build Array (concatenate)(w5868, w5855) -> (w5867:dbl[])
                n3772 = Select(t=w5855, s=w5787, f=w5867) -> (s? t:f=w5842:dbl[])
                n3773 = feedback-in #32(w5842) -> ()
                n3774 = Divide(x=w5882, y=w5883) -> (x/y=w5885:dbl)
                n3775 = Multiply(x=w5885, y=100.0) -> (x*y=w5884:dbl)
                n3776 = Build Array(w5842, w5837, w5798) -> (→"Saved APD":dbl[][])
                n3777 = Array Size(array=w5842) -> (size(s)=w5860:i32)
                n3778 = Unbundle By Name(w5862) -> ("Y"=w5866:dbl[])
                n3779 = Subtract(x=w5860, y="N pts to average") -> (x-y=w5795:i32)
                n3780 = Multiply(x="N pts to average", y=u16 2) -> (x*y=w5838:u16)
                n3781 = Subtract(x=w5860, y=w5838) -> (x-y=w5796:i32)
                n3782 = feedback #33(w5866) -> (w5865:dbl[])
                n3783 = Build Array (concatenate)(w5865, w5866) -> (w5864:dbl[])
                n3784 = Select(t=w5866, s=w5787, f=w5864) -> (s? t:f=w5863:dbl[])
                "Trap Delta Graph" <- w5863
                n3785 = feedback-in #33(w5863) -> ()
                n3786 = Array Subset(array=w5842, index=w5795, length="N pts to average") -> (w5859:dbl[])
                n3787 = Array Subset(array=w5842, index=w5796, length="N pts to average") -> (w5858:dbl[])
                n3788 = Array Subset(array=w5837, index=w5795, length="N pts to average") -> (w5840:dbl[])
                n3789 = Array Subset(array=w5837, index=w5796, length="N pts to average") -> (w5839:dbl[])
                n3790 = Array Subset(array=w5798, index=w5795, length="N pts to average") -> (w5807:dbl[])
                n3791 = Array Subset(array=w5798, index=w5796, length="N pts to average") -> (w5806:dbl[])
                n3792 = Index Array(array=w5820, index=0) -> (element=w5818:waveform(dbl))
                n3793 = call-poly <vilib>:"Mean.vi"("X"=w5859) -> ("mean"=w5857:dbl)  [unwired: 1 out]
                n3794 = call-poly <vilib>:"Mean.vi"("X"=w5840) -> ("mean"=w5836:dbl)  [unwired: 1 out]
                n3795 = call-poly <vilib>:"Mean.vi"("X"=w5858) -> ("mean"=w5856:dbl)  [unwired: 1 out]
                n3796 = call-poly <vilib>:"Mean.vi"("X"=w5839) -> ("mean"=w5835:dbl)  [unwired: 1 out]
                n3797 = call-poly <vilib>:"Mean.vi"("X"=w5807) -> ("mean"=w5805:dbl)  [unwired: 1 out]
                n3798 = call-poly <vilib>:"Mean.vi"("X"=w5806) -> ("mean"=w5804:dbl)  [unwired: 1 out]
                n3799 = Unbundle By Name(w5818) -> ("Y"=w5816:dbl[])
                n3800 = Subtract(x=w5836, y=w5835) -> (x-y=w5827:dbl)
                "Delta Fl. 2" <- w5827
                n3801 = Subtract(x=w5805, y=w5804) -> (x-y=w5799:dbl)
                "Delta Fl. 3" <- w5799
                n3802 = Subtract(x=w5857, y=w5856) -> (x-y=w5854:dbl)
                "Delta Fl. 1" <- w5854
                n3803 = feedback #34(w5816) -> (w5815:dbl[])
                n3804 = Build Array (concatenate)(w5815, w5816) -> (w5817:dbl[])
                n3805 = Initialize Array(w5854, 1 ("dimension size")) -> (w5851:dbl[])
                n3806 = Initialize Array(w5827, 1 ("dimension size")) -> (w5832:dbl[])
                n3807 = Initialize Array(w5799, 1 ("dimension size")) -> (w5801:dbl[])
                n3808 = Select(t=w5816, s=w5787, f=w5817) -> (s? t:f=w5814:dbl[])
                "Saved trap pos" <- w5814
                n3809 = feedback-in #34(w5814) -> ()
                n3810 = feedback #35(w5851) -> (w5852:dbl[])
                n3811 = Build Array (concatenate)(w5852, w5851) -> (w5850:dbl[])
                n3812 = feedback #36(w5832) -> (w5833:dbl[])
                n3813 = feedback #37(w5801) -> (w5802:dbl[])
                n3814 = Build Array (concatenate)(w5833, w5832) -> (w5831:dbl[])
                n3815 = Build Array (concatenate)(w5802, w5801) -> (w5800:dbl[])
                n3816 = Select(t=w5851, s=w5787, f=w5850) -> (s? t:f=w5830:dbl[])
                n3817 = feedback-in #35(w5830) -> ()
                n3818 = Select(t=w5832, s=w5787, f=w5831) -> (s? t:f=w5829:dbl[])
                n3819 = feedback-in #36(w5829) -> ()
                n3820 = Select(t=w5801, s=w5787, f=w5800) -> (s? t:f=w5794:dbl[])
                n3821 = feedback-in #37(w5794) -> ()
                n3822 = Build Array(w5830, w5829, w5794) -> (→"Save APD Deriv":dbl[][])
                n3823 = Index Array(array=w5786, index=15) -> (element=w5792:waveform(dbl))
                n3824 = Unbundle By Name(w5792) -> ("Y"=w5790:dbl[])
                n3825 = feedback #38(w5790) -> (w5789:dbl[])
                n3826 = Build Array (concatenate)(w5789, w5790) -> (w5791:dbl[])
                n3827 = Select(t=w5790, s=w5787, f=w5791) -> (s? t:f=w5788:dbl[])
                "Amp current" <- w5788
                n3828 = feedback-in #38(w5788) -> ()
              }
            }
            "Progress" <- w5763
            "Progress 2" <- w5763
          }
        }
      }
    }
    n3829 = local read "wait to reset values"() -> (w4576:bool)
    n3830 = Not(x=w4574) -> (.not. x?=w4577:bool)
    n3831 = And(x=w4577, y=w4576) -> (x .and. y?=w4578:bool)
    n3832 = case "Part of MCL raster scanning: returns to initial positions after scan done" shown="True" w4578 {
      tunnel: w4325 -> [w5226 w5233]
      tunnel: [w5226 w5232] -> w4580
      tunnel: w4425 -> [w5225 w5231]
      tunnel: [w5225 w5230] -> w4575
      frame False {
      }
      frame True {
        w5241 = 10.0 ("y")
        w5240 = 32767.0 ("y")
        # "to return scan values\nafter a synchronous \nAOM scan"
        n3833 = local read "AO2"() -> (w5234:dbl)
        n3834 = local read "AO1"() -> (w5235:dbl)
        n3835 = local write "wait to reset values"(FALSE ("wait to reset values")) -> ()
        n3836 = Multiply(x=w5235, y=w5240) -> (x*y=w5237:dbl)
        n3837 = Multiply(x=w5234, y=w5240) -> (x*y=w5239:dbl)
        n3838 = Divide(x=w5237, y=w5241) -> (x/y=w5236:dbl)
        n3839 = Divide(x=w5239, y=w5241) -> (x/y=w5238:dbl)
        n3840 = To Word Integer(number=w5236) -> (16bit integer=w5242:i16)
        n3841 = To Word Integer(number=w5238) -> (16bit integer=w5243:i16)
        n3842 = local read "Total Counts (ticks)"() -> (w5227:u16)
        n3843 = local read "Scan Range (V)\n(of steps)"() -> (w5228:dbl)
        n3844 = xnode "Read/Write Control"("FPGA VI Reference In"=w5233, "error in"=w5231, "AO1 (Y)"=w5242, "AO2 (X)"=w5243, "MCL count"=w5227) -> ("FPGA VI Reference Out"=w5232:T41, "error out"=w5230:errorcluster)
        n3845 = property on="Scan Range (V)\n(of steps)" class="DigNum (strict)"("Val(Sgnl)"=w5228) -> ()  [unwired: 2 in, 2 out]
      }
    }
    n3846 = case shown="True" "Sound ON" {
      tunnel: [w4691 w4736] -> w4377
      tunnel: w4376 -> [w4691 w4735]
      tunnel: w4374 -> [_ _]
      tunnel: w4354 -> [_ w4694]
      tunnel: w4373 -> [_ _]
      tunnel: w4372 -> [_ w4705]
      tunnel: w4371 -> [_ w4715]
      frame False {
      }
      frame True {
        n3847 = Index Array(array=w4694, index="Data channel to sound") -> (element=w4693:waveform(dbl))
        "Waveform Graph 2" <- w4693
        n3848 = Unbundle By Name(w4693) -> ("dt"=w4719:dbl, "Y"=w4717:dbl[])
        n3849 = Array Size(array=w4717) -> (size(s)=w4718:i32)
        "N data samples" <- w4718
        n3850 = for "Data time base" {
          N: w4718 -> [_]
          tunnel: [w4740] -> w4720 mode=indexing
          i -> [w4740]
        }
        n3851 = Multiply(x=w4719, y=w4720) -> (x*y=w4716:dbl[])
        n3852 = Compound Arithmetic op=MULTIPLY(6.283185307179586, "Carrier Frequency (Hz)", w4715) -> (w4732:dbl[])
        n3853 = call <vilib>:"Interpolate 1D.vi"("X is monotonic"=TRUE, "xi"=w4715, "X"=w4716, "Y"=w4717) -> ("yi"=w4713:dbl[])  [unwired: 5 in, 2 out]
        n3854 = Sine(x=w4732) -> (sin(x)=w4721:dbl[])
        n3855 = Add(x=w4713, y="Offset") -> (x+y=w4711:dbl[])
        n3856 = Multiply(x=w4711, y="mult x") -> (x*y=w4709:dbl[])
        n3857 = Add(x="Offset 2", y=w4709) -> (x+y=w4704:dbl[])
        n3858 = Compound Arithmetic op=MULTIPLY(6.283185307179586, "Carrier Frequency (Hz)", w4705, w4704) -> (w4696:dbl[])
        n3859 = for "Cumulative sum" {
          tunnel: [w4739] -> w4702 mode=indexing
          shift-right: [w4739] -> w4699
          shift-left: 0.0 -> [w4738]
          tunnel: w4696 -> [w4737] mode=indexing
          n3860 = Add(x=w4737, y=w4738) -> (x+y=w4739:dbl)
        }
        n3861 = feedback #39(0.0) -> (w4698:dbl)
        n3862 = Add(x=w4702, y=w4698) -> (x+y=w4701:dbl[])
        n3863 = Add(x=w4699, y=w4698) -> (x+y=w4697:dbl)
        n3864 = feedback-in #39(w4697) -> ()
        n3865 = Sine(x=w4701) -> (sin(x)=w4695:dbl[])
        n3866 = Select(t=w4721, s="tone or data", f=w4695) -> (s? t:f=w4727:dbl[])
        n3867 = Multiply(x=w4727, y="Volume") -> (x*y=w4725:dbl[])
        n3868 = Initialize Array(0.0 ("element"), "N initial buffer elements") -> (w4728:dbl[])
        n3869 = Multiply(x="N initial buffer elements", y=w4705) -> (x*y=→"Initial buffer time (s)":dbl)
        n3870 = Build Array (concatenate)(w4728, w4725) -> (w4730:dbl[])
        n3871 = First Call?() -> (First Call?: T/F=w4731:bool)
        n3872 = Select(t=w4730, s=w4731, f=w4725) -> (s? t:f=w4724:dbl[])
        n3873 = call-poly <vilib>:"Sound Output Write.vi"("data"=w4724, "task ID"=w4735) -> ("task ID out"=w4736:T52)  [unwired: 8 in, 1 out]
      }
    }
    n3874 = node-c288() -> ()  [unwired: 2 out]
  }
  n3875 = disable-structure shown="Disabled" {
    disable-tunnel: w20 -> [w5931 _]
    frame Disabled {
      n3876 = call <vilib>:"Sound Output Clear.vi"("task ID"=w5931) -> ()  [unwired: 10 in, 1 out]
    }
    frame Enabled {
    }
  }
  n3877 = node-c288(w62) -> ()  [unwired: 1 out]
  n3878 = node-c288(w70) -> ()  [unwired: 1 out]
  n3879 = flat-sequence {
    tunnel: w77 -> [w5935]
    tunnel: w78 -> [w5936]
    tunnel: [w5934] -> w76
    tunnel: [w5933] -> w75
    tunnel: w74 -> [_]
    tunnel: w72 -> [_]
    tunnel: w68 -> [_]
    tunnel: w76 -> [w5937]
    tunnel: w75 -> [w5938]
    frame #0 {
      w5932 = FALSE ("AI to FIFO")
      n3880 = xnode "Read/Write Control"("FPGA VI Reference In"=w5936, "error in"=w5935, "AI to FIFO"=w5932, "APD to FIFO"=w5932) -> ("FPGA VI Reference Out"=w5934:T41, "error out"=w5933:errorcluster)
    }
    frame #1 {
      n3881 = xnode "Close FPGA VI Reference"("FPGA VI Reference In"=w5937, "error in"=w5938) -> ("error out"=→"error out":errorcluster)
    }
  }
